vi "MPS_main.vi"() -> ()   [LabVIEW 2021] (continued)
  out "Numeric":i32
  out "Recent File Name":string="MAG_Empty_0,0000010_ug_BatchName"
  in  "name identifier":string="Empty"
  in  "Base path":path=path "D:/HumanImagerData/MPS Data"
  out "Meas Drive IMon Val RMS\nCal BMon":dbl=0.07740384925739274
  in  "Acq Baseline":bool
  in  "CalcConc":bool
  in  "CalcMass":bool
  in  "Sample MetaData Cluster":T1={"Sample Volume (uL)"=10.0, "Sample Mass (ug)"=1e-06, "Sample Conc(mg/mL)"=1e-07, "Sample Temperature (C)"=23.0, "Batch Num"=222.0, "Batch Name"="BatchName", "Solute"="Test", "Solvent"="Water", "Sample Description"="EMPTY"}
  in  "TxRx_Params":T2={"sample rate"=1000000.0, "Tx freq"=23809.52380952381, "Tx amp"=0.05, "Tx cycles\nSpectroscopy"=500.0, "Bias amp"=2.65, "Bias freq"=11.904761904761905, "Receive range"=5.0, "Bias Periods\nMagnetometry"=6.0, "Tx Freq Division Factor"=42.0, "Drive Periods per Bias"=2000.0, "TX harmonics"=[47619.04761904762, 71428.57142857142, 95238.09523809524, 119047.61904761905, 142857.14285714284, 166666.66666666666, 190476.19047619047, 214285.7142857143, 238095.2380952381, 261904.7619047619, 285714.2857142857, 309523.8095238095, 333333.3333333333, 357142.85714285716, 380952.38095238095, 404761.90476190473, 428571.4285714286, 452380.95238095237, 476190.4761904762, 500000.0]} {"TX harmonics" format="%#_6p"}
  in  "Tab Control 2":enum32{"Motor Params", "Motor Move Control"}(tab)=enum."Motor Move Control"
  out "Motor Dir\nT=Fwd":bool=TRUE
  in  "pulse duration (T/2)":dbl=0.0005 format="%#_13p"
  in  "Motor speed":string(combo)="Sixteenth step"
  in  "Sequence to run on start up":string[](array[string])=["Move", "Halt"]
  out "Current Motor State":string="MoveToMax"
  in  "Unsigned Pulses to move":dbl=5.0
  in  "Move-Bed-Back":bool
  in  "Move-Bed-Fwd":bool
  in  "Home then insert sample":bool
  in  "Pulses From Home to Max Sig":dbl=128.0
  in  "Motor Go Home":bool
  out "Empty Bore-BMon-Spec":dbl[](array[numeric])
  out "EmptyBoreBaseline_Mag_BMon":dbl[](array[numeric])
  in  "Toggle fan":bool
  out "Amps Drive Peak":dbl=13.682895644634083
  out "EmptyBoreBaseline_Mag":dbl[](array[numeric])
  out "Samples Per Acquisition":dbl=504000.0
  in  "Run Cal BMon":bool
  out "mT/BMon Volt":dbl=19.366390338753
  out "Meas BMon Val RMS":dbl=0.4592431533931806
  out "Expected mT peak":dbl=8.893882169012155
  in  "Update global variables Button":bool
  in  "stop":bool
  out "current system state":string="Idle"
  out "Main loop has stopped":bool
  in  "Tab Control":T3(tab)=enum."Magnetometry"
  in  "Run Sys Ref Meas":bool
  in  "Use Bias?":bool
  in  "Scanner Description":T4={"Scanner Name"="Test", "Hardware description"="Test", "Preamplifier Used"="INA", "Preamp Gain"=9999.0, "Drive Amplifier"="TDA3255", "Bias Amplifier"="RCF IPS700", "Drive Current Monitor"="Rogowski", "Bias Current Monitor"="ACS-770"}
  in  "Study and Experiment Description":T5={"Study Number"=9999, "Study Name"="Test", "UUID"="93C38C5B-0D33-4591-A951-706E1E8CC347", "GUI Open Time"="2022-04-10_16-04-30", "Notes"="Example"}
  out "3f0 over time":dbl(graph)=3.5778765993993083e-09
  out "Rx FFT":cluster{"f0":dbl, "df":dbl, "magnitude":dbl[]}(graph)={"f0"=0.0, "df"=49.55401387512537, "magnitude"=array[10090 elements]}
  in  "Run Spectroscopy":bool
  in  "Stop Spec":bool
  out "Loop Num":i32=5 format="%.4p"
  in  "Save Spectroscopy":bool=TRUE
  in  "Max Spec Runs":i32=10000
  in  "ms delay":u32=25 format="%#.4p"
  in  "Spec samples\nto crop":dbl=820.0 format="%#_4p"
  out "Spec Time Domain":dbl[][](graph)
  out "f0 over time":dbl(graph)=4.148276400287791e-05
  out "THD":dbl=-79.42517157036677 format="%#_6p"
  out "Expected mT Spec Drive":dbl=9.011999624680417 format="%#_4p"
  out "mean3f0":dbl=3.083839308845972e-09 format="%#_3p"
  out "standard deviation 3f0":dbl=4.1440630531044285e-10 format="%#_4p"
  out "meanf0":dbl=4.1403379240994345e-05 format="%#_3p"
  out "standard deviation f0":dbl=8.05138622723974e-08 format="%#_4p"
  out "Bed moving":bool=TRUE
  in  "ms delay\nevery Spec":u32=50 format="%#.4p"
  in  "Run in-out spec":bool
  out "Expected mT Spec Drive 2":dbl=9.006191537419065 format="%#_4p"
  out "Drive Imon THD 2":dbl=-79.0246761592133 format="%#_6p"
  in  "Spec samples\nto crop_InOut":dbl=820.0 format="%#_4p"
  out "3f0 over time 2":dbl(graph)=9.016336929462854e-10
  out "f0 over time 2":dbl(graph)=6.340842124732096e-07
  out "Loop Num 2":i32=6 format="%.4p"
  out "Spec Time Domain 2":dbl[][](graph)
  out "Rx FFT 2":cluster{"f0":dbl, "df":dbl, "magnitude":dbl[]}(graph)={"f0"=0.0, "df"=49.55401387512537, "magnitude"=array[10090 elements]}
  in  "Num acq per\ncycle":i32=6
  in  "Save Spectroscopy 2":bool=TRUE
  in  "Number of cycles":i32=5
  in  "Pulses in/out":dbl=50.0
  out "Run number":i32=70
  in  "Run Mag":bool
  out "Susceptibility Curves":cluster{"Y":dbl[], "Y":dbl[]}[](graph)
  in  "Save Mag data":bool
  out "Rx Smooth":dbl[](graph)
  out "Sensitivity profile":dbl[][](graph)
  in  "Num Mag Avgs":i32=1 min=1
  out "RunNum":i32
  in  "Pulses in/out 2":dbl=50.0
  in  "ms delay each run":u32
  out "Sample Out":bool
  out "RxEmptyBore-Mag":waveform(dbl)(graph)={"t0"=timestamp(3732466214.765835 s since 1904-01-01), "dt"=9.9999999999997e-07, "Y"=array[504000 elements], "attributes"=variant("NI_ChannelName"=variant(string "H1/ai7"), "NI_UnitDescription"=variant(string "Volts"))}
  out "EmptyBoreBaseline_Spec":dbl[](array[numeric])
  out "RxEmptyBore-Spec":dbl[](graph)
  out "3f0 vs Mass":T6(graph)
  in  "Run DilutionAdd":bool
  in  "ms delay 2":u32=25 format="%#.4p"
  in  "File Name Dilution":string="450ng_Syno"
  in  "Base path 4":path=path "D:/HumanImagerData/MPS Data"
  out "Expected mT Spec Drive 3":dbl=7.493132421986184 format="%#_4p"
  out "THD 2":dbl=-78.20284195000295 format="%#_6p"
  in  "Spec samples\nto crop 3":dbl=820.0 format="%#_4p"
  in  "Num Dil Series Runs":i32=7
  in  "Clear Dilution Array":bool
  out "r^2":dbl format="%.4f"
  in  "Delete Last Meas":bool
  out "Dilution Array\nConc,f0,f3":dbl[][](array[numeric])
  in  "Save Dilution Array":bool
  # "MPS"
  # "FILE SAVING"
  # "NOT WORKING YET"
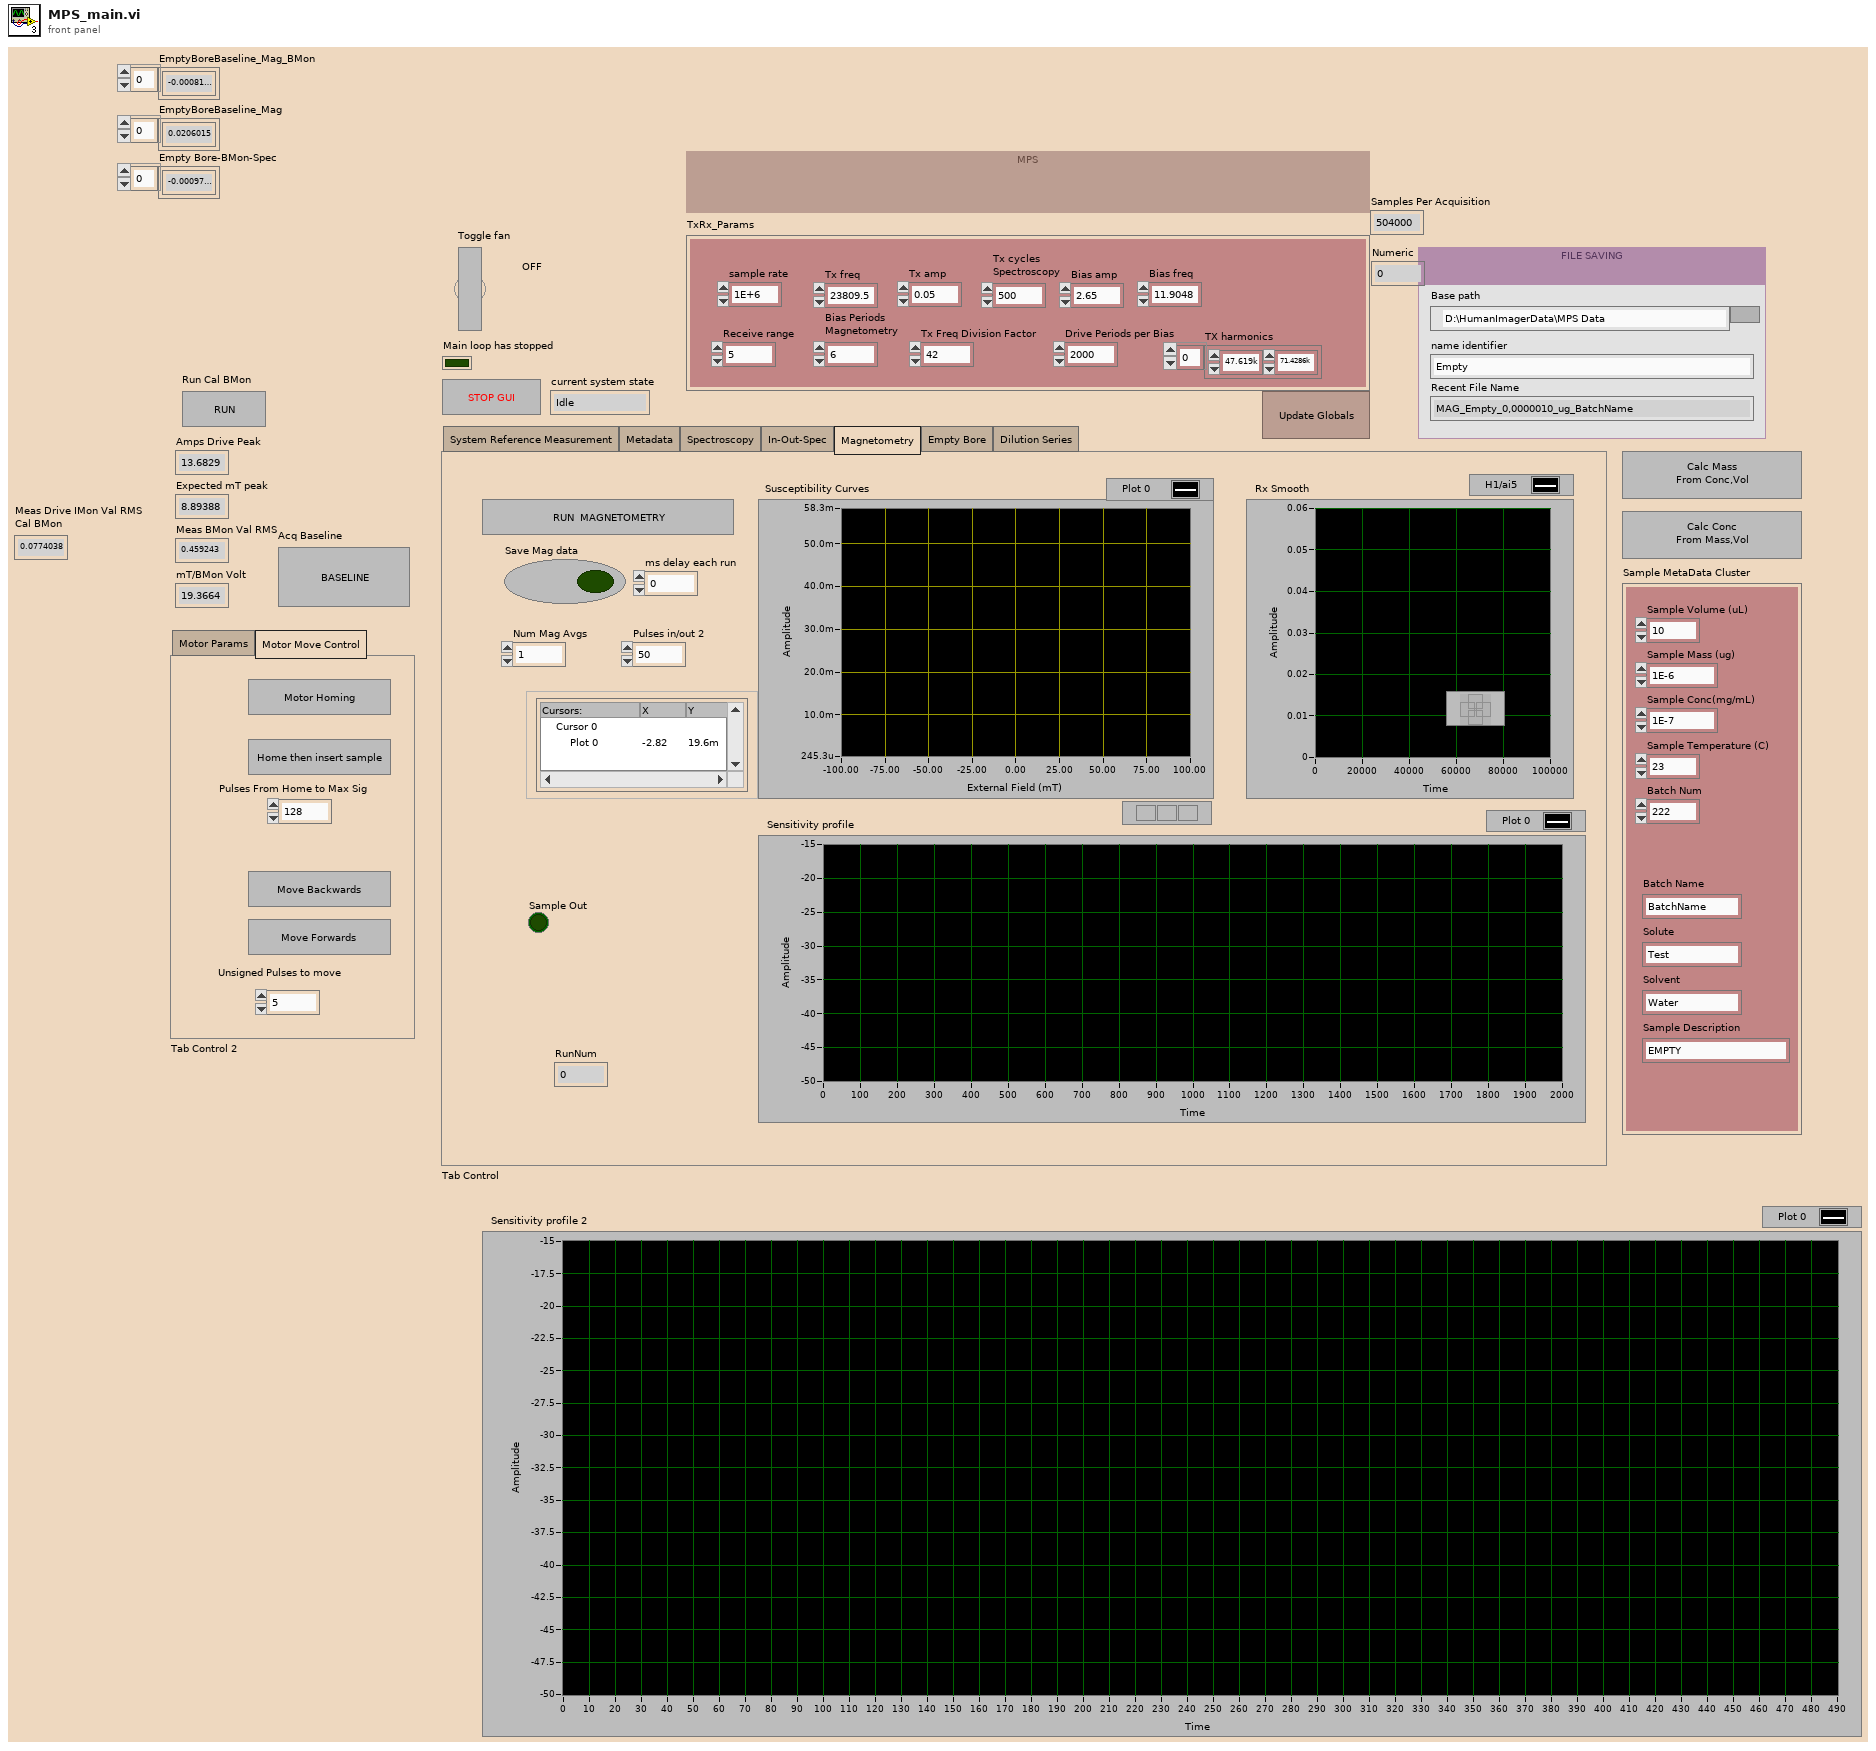
[diagram p1: front panel]
types:
  T1 = cluster{"Sample Volume (uL)":dbl, "Sample Mass (ug)":dbl, "Sample Conc(mg/mL)":dbl, "Sample Temperature (C)":dbl, "Batch Num":dbl, "Batch Name":string, "Solute":string, "Solvent":string, "Sample Description":string}
  T2 = cluster{"sample rate":dbl, "Tx freq":dbl, "Tx amp":dbl, "Tx cycles\nSpectroscopy":dbl, "Bias amp":dbl, "Bias freq":dbl, "Receive range":dbl, "Bias Periods\nMagnetometry":dbl, "Tx Freq Division Factor":dbl, "Drive Periods per Bias":dbl, "TX harmonics":dbl[]}
  T3 = enum32{"System Reference Measurement", "Metadata", "Spectroscopy", "In-Out-Spec", "Magnetometry", "Empty Bore", "Dilution Series"}
  T4 = cluster{"Scanner Name":string, "Hardware description":string, "Preamplifier Used":string, "Preamp Gain":dbl, "Drive Amplifier":string, "Bias Amplifier":string, "Drive Current Monitor":string, "Bias Current Monitor":string}
  T5 = cluster{"Study Number":i64, "Study Name":string, "UUID":string, "GUI Open Time":string, "Notes":string}
  T6 = cluster{"Dilution Array\nConc,f0,f3":dbl[], "Dilution Array\nConc,f0,f3":dbl[]}[]
  T7 = cluster{"sample rate":dbl, "Transmit frequency":dbl, "Transmit amplitude":dbl, "sample rate digital out":dbl, "TX cycles":i32, "sample rate DAQ1":dbl, "Receive frequency":dbl, "Receive range":dbl, "TX harmonics":dbl[]}
  T8 = cluster{"Drive IMon":dbl[], "Rx Time Domain":dbl[], "Rx Empty Bore":dbl[], "BMon":dbl[], "Bias IMon":dbl[], "TF-Corr-MagOverTime":dbl[], "Interpolated Rx TF-Mag":dbl[], "Interpolated Rx TF-Phase":dbl[]}
  T9 = cluster{"slope min":dbl, "slope max":dbl, "intercept min":dbl, "intercept max":dbl}
  T10 = enum32{"none", "input signal", "detected signal", "residual signal"}
  T11 = typedef "NI_AALPro.lvlib/windowTd.ctl" = u32
  T12 = typedef "Tag-dbl.lvlib/))Channel.ctl" = refnum<queue>
  T13 = cluster{"Dilution Array\nConc,f0,f3":dbl[], "Dilution Array\nConc,f0,f3":dbl[]}
  T14 = cluster{"Dilution Array\nConc,f0,f3":dbl[], "Best Linear Fit":dbl[]}
  T15 = cluster{"exported time signal":waveform(dbl), "exported spectrum (dB)":cluster{"f0":dbl, "df":dbl, "dB Spectrum (Hann)":dbl[]}}
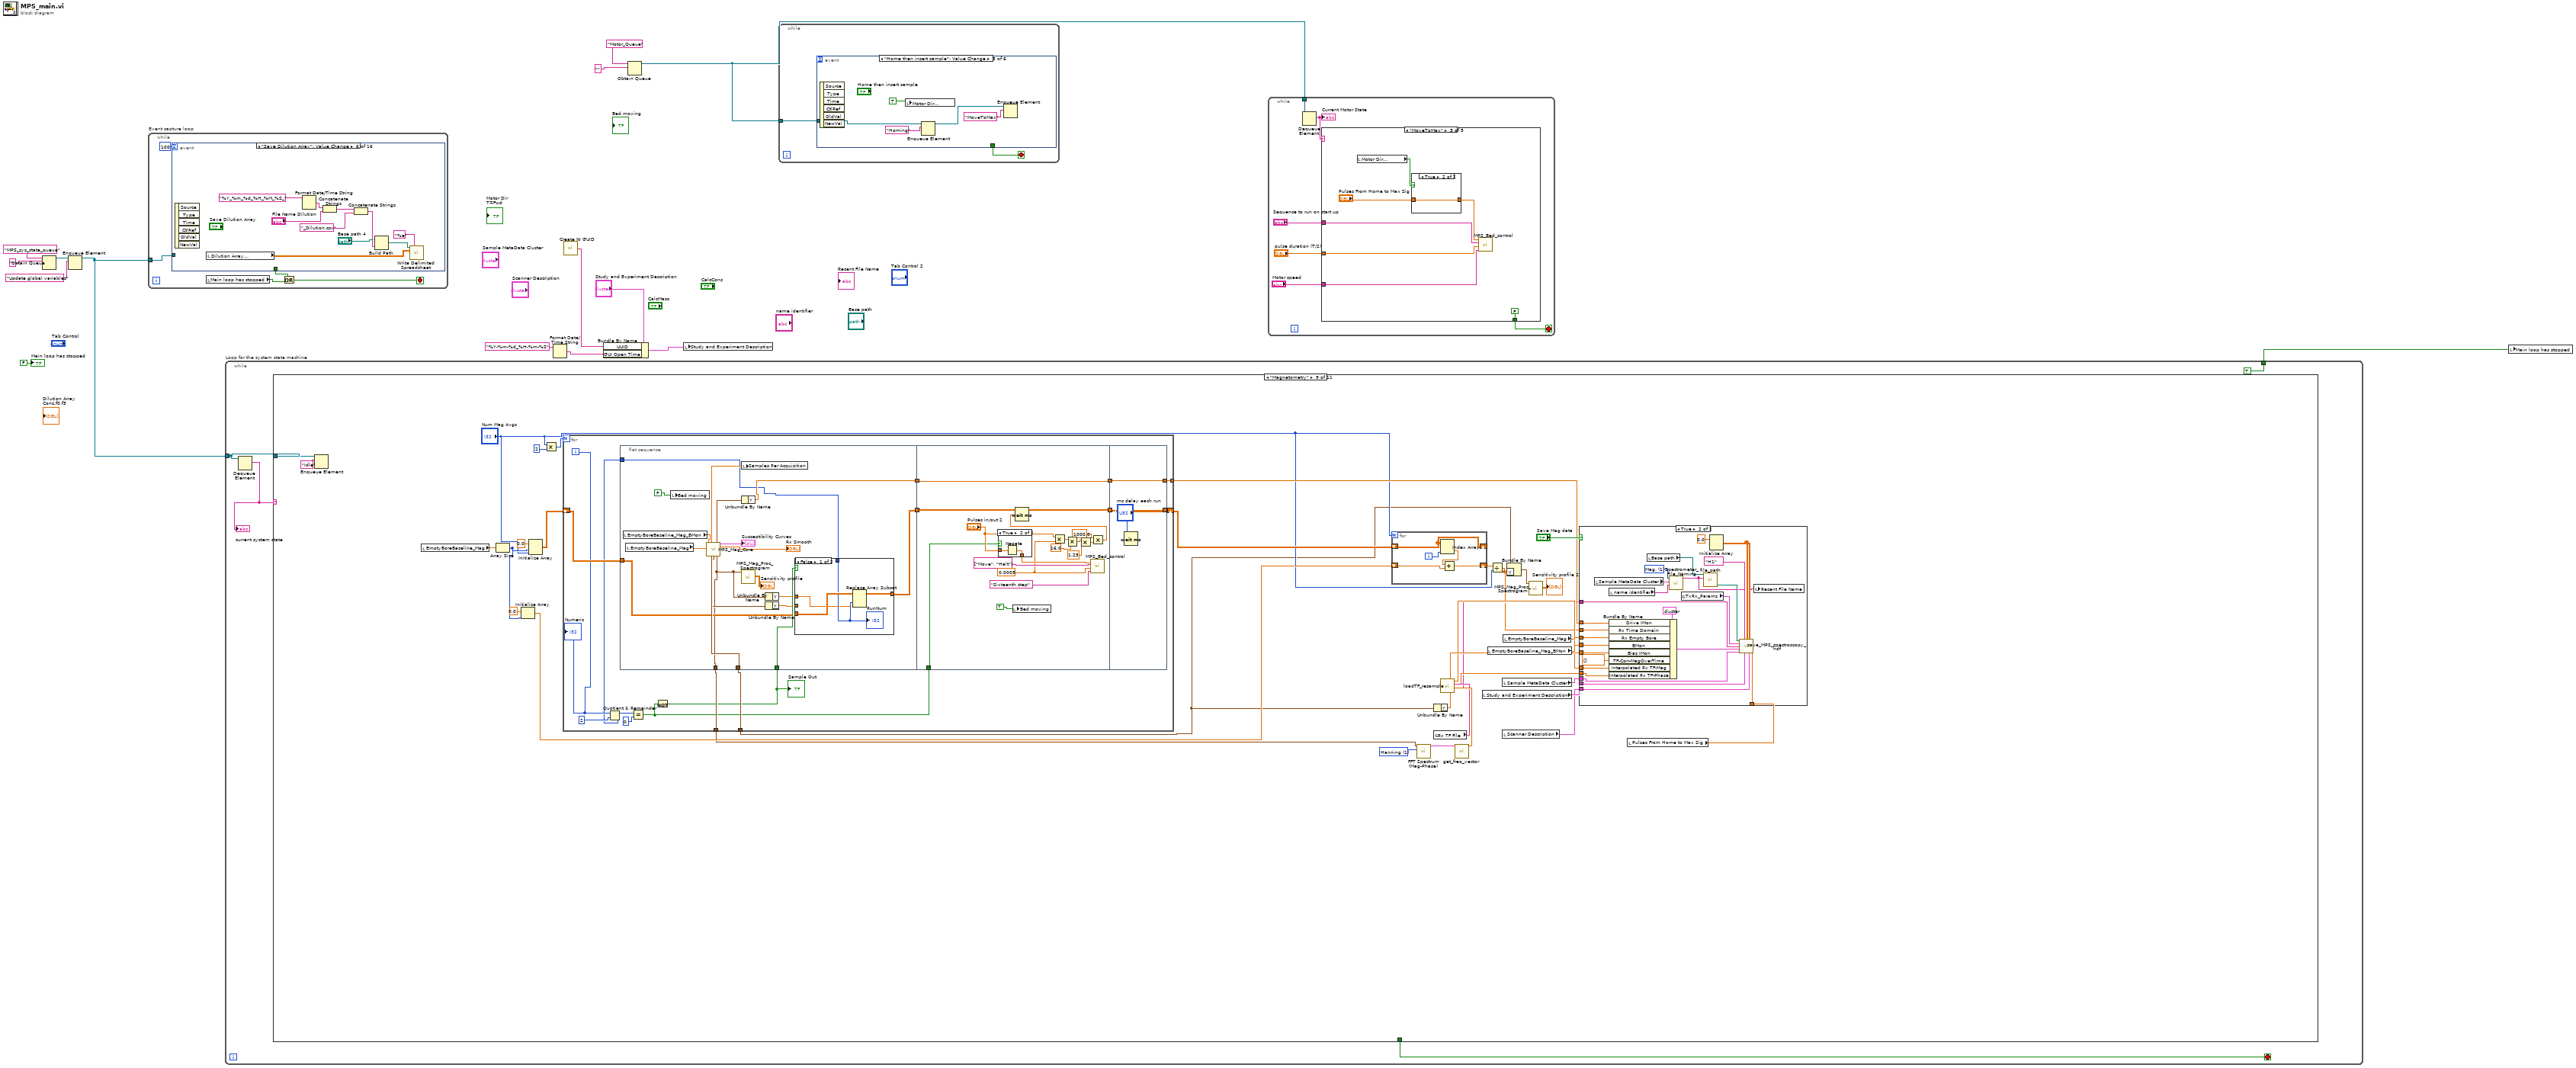
[diagram p0: block diagram]
diagram:
  n1 = Obtain Queue(name (unnamed)="MPS_sys_state_queue", element data type="") -> (queue out=w11:refnum<queue>)  [unwired: 3 in, 2 out]
  n2 = Enqueue Element(queue=w11, element="Update global variables") -> (queue out=w9:refnum<queue>)  [unwired: 2 in, 2 out]
  n3 = while "Event capture loop" {
    tunnel: w9 -> [w19]
    stop <- w16 stop-if-true
    n4 = event shown="[5] \"Save Dilution Array\": Value Change" {
      selector: _ -> [_ _ _ _ _ _ _ _ _ _ _ _ _ _ _ _]
      dyn-events: _ -> [_ _ _ _ _ _ _ _ _ _ _ _ _ _ _ _]
      timeout: 100 -> [_ _ _ _ _ _ _ _ _ _ _ _ _ _ _ _]
      tunnel: w19 -> [_ w22 w24 w26 _ _ _ w66 w68 w70 w72 _ _ _ w93 w96]
      tunnel: [FALSE ("x") _ _ _ _ _ _ _ _ _ _ _ _ _ _ TRUE ("x")] -> w17
      event Timeout {
        n5 = event-data() -> ()  [unwired: 1 in, 3 out]
      }
      event "Run Sys Ref Meas": Value Change {
        n6 = event-data() -> ()  [unwired: 1 in, 6 out]
        n7 = Enqueue Element(queue=w22, element="System Reference Measurement") -> ()  [unwired: 2 in, 3 out]
      }
      event "Run Spectroscopy": Value Change {
        n8 = event-data() -> ()  [unwired: 1 in, 6 out]
        n9 = Enqueue Element(queue=w24, element="Spectroscopy") -> ()  [unwired: 2 in, 3 out]
      }
      event "Run DilutionAdd": Value Change {
        n10 = event-data() -> ()  [unwired: 1 in, 6 out]
        n11 = Enqueue Element(queue=w26, element="Acquire Dilution Data") -> ()  [unwired: 2 in, 3 out]
      }
      event "Clear Dilution Array": Value Change {
        n12 = event-data() -> ()  [unwired: 1 in, 6 out]
        n13 = Initialize Array(0.0 ("element"), 0 ("dimension size"), 3 ("dimension size")) -> (w28:dbl[][])
        n14 = local write "Dilution Array\nConc,f0,f3"(w28) -> ()
        n15 = Index Array(array=w28, index (col)=0 ("disabled index (col)")) -> (element=w35:dbl[])  [unwired: 1 in]
        n16 = Index Array(array=w28, index (col)=2 ("disabled index (col)")) -> (element=w36:dbl[])  [unwired: 1 in]
        n17 = call <vilib>:"Linear Fit.vi"("Y"=w36, "X"=w35) -> ("Best Linear Fit"=w34:dbl[])  [unwired: 9 in, 4 out]
        n18 = Bundle(w35, w36) -> (w32:cluster{dbl[], dbl[]})  [unwired: 1 in]
        n19 = call <vilib>:"Correlation Coefficient (Spearman).vi"("Y"=w36, "X"=w35) -> ()  [unwired: 8 in, 2 out]
        n20 = Bundle(w35, "Best Linear Fit"=w34) -> (w33:cluster{dbl[], "Best Linear Fit":dbl[]})  [unwired: 1 in]
        n21 = Build Array(w33, w32) -> (w31:cluster{dbl[], "Best Linear Fit":dbl[]}[])
        n22 = local write "3f0 vs Mass"(w31) -> ()
      }
      event "Save Dilution Array": Value Change {
        n23 = event-data() -> ()  [unwired: 1 in, 6 out]
        n24 = local read "Dilution Array\nConc,f0,f3"() -> (w41:dbl[][])
        n25 = Format Date/Time String(time format string (%c)="%Y_%m_%d_%H_%M_%S_") -> (date/time string=w47:string)  [unwired: 2 in]
        n26 = Concatenate Strings(w47, "File Name Dilution") -> (w49:string)
        n27 = Concatenate Strings(w49, "_Dilution.csv" ("string")) -> (w48:string)
        n28 = Build Path(base path="Base path 4", name or relative path=w48) -> (appended path=w42:path)
        n29 = call-poly <vilib>:"Write Delimited Spreadsheet.vi"("file path (dialog if empty)"=w42, "format (%.3f)"="%e", "2D data"=w41) -> ()  [unwired: 11 in, 2 out]
      }
      event "Delete Last Meas": Value Change {
        n30 = event-data() -> ()  [unwired: 1 in, 6 out]
        n31 = local read "Dilution Array\nConc,f0,f3"() -> (w65:dbl[][])
        n32 = Array Size(array=w65) -> (size(s)=w64:i32[])
        n33 = Index Array(array=w64, index=0) -> (element=w62:i32)
        n34 = Decrement(x=w62) -> (x-1=w61:i32)
        n35 = Array Subset(array=w65, index (row)=0 ("index"), length (row)=w61, index (col)=0 ("index")) -> (w51:dbl[][])  [unwired: 1 in]
        n36 = local write "Dilution Array\nConc,f0,f3"(w51) -> ()
        n37 = Index Array(array=w51, index (col)=0 ("disabled index (col)")) -> (element=w57:dbl[])  [unwired: 1 in]
        n38 = Index Array(array=w51, index (col)=2 ("disabled index (col)")) -> (element=w58:dbl[])  [unwired: 1 in]
        n39 = call <vilib>:"Linear Fit.vi"("Y"=w58, "X"=w57) -> ("Best Linear Fit"=w56:dbl[])  [unwired: 9 in, 4 out]
        n40 = Bundle(w57, w58) -> (w54:cluster{dbl[], dbl[]})  [unwired: 1 in]
        n41 = call <vilib>:"Correlation Coefficient (Spearman).vi"("Y"=w58, "X"=w57) -> ()  [unwired: 8 in, 2 out]
        n42 = Bundle(w57, "Best Linear Fit"=w56) -> (w55:cluster{dbl[], "Best Linear Fit":dbl[]})  [unwired: 1 in]
        n43 = Build Array(w55, w54) -> (w50:cluster{dbl[], "Best Linear Fit":dbl[]}[])
        n44 = local write "3f0 vs Mass"(w50) -> ()
      }
      event "Run in-out spec": Value Change {
        n45 = event-data() -> ()  [unwired: 1 in, 6 out]
        n46 = Enqueue Element(queue=w66, element="In-Out-Spec") -> ()  [unwired: 2 in, 3 out]
      }
      event "Run Mag": Value Change {
        n47 = event-data() -> ()  [unwired: 1 in, 6 out]
        n48 = Enqueue Element(queue=w68, element="Magnetometry") -> ()  [unwired: 2 in, 3 out]
      }
      event "Acq Baseline": Value Change {
        n49 = event-data() -> ()  [unwired: 1 in, 6 out]
        n50 = Enqueue Element(queue=w70, element="Acquire Empty Bore") -> ()  [unwired: 2 in, 3 out]
      }
      event "Run Cal BMon": Value Change {
        n51 = event-data() -> ()  [unwired: 1 in, 6 out]
        n52 = Enqueue Element(queue=w72, element="Cal_BMon") -> ()  [unwired: 2 in, 3 out]
      }
      event "CalcMass": Value Change {
        n53 = event-data() -> ()  [unwired: 1 in, 6 out]
        n54 = local read "Sample MetaData Cluster"() -> (w78:T1)
        n55 = Unbundle By Name(w78) -> ("Sample Volume (uL)"=w77:dbl, "Sample Conc(mg/mL)"=w76:dbl)
        n56 = Multiply(x=w77, y=w76) -> (x*y=w74:dbl)
        n57 = Bundle By Name(cluster=w78, "Sample Mass (ug)"=w74) -> (w75:T1)
        n58 = local write "Sample MetaData Cluster"(w75) -> ()
      }
      event "CalcConc": Value Change {
        n59 = event-data() -> ()  [unwired: 1 in, 6 out]
        n60 = local read "Sample MetaData Cluster"() -> (w83:T1)
        n61 = Unbundle By Name(w83) -> ("Sample Mass (ug)"=w82:dbl, "Sample Volume (uL)"=w81:dbl)
        n62 = Divide(x=w82, y=w81) -> (x/y=w79:dbl)
        n63 = Bundle By Name(cluster=w83, "Sample Conc(mg/mL)"=w79) -> (w80:T1)
        n64 = local write "Sample MetaData Cluster"(w80) -> ()
      }
      event "Toggle fan": Value Change {
        n65 = event-data() -> ()  [unwired: 1 in, 6 out]
        n66 = global read "MPS_global_variables.vi" "Fan Control Line"() -> (w88:tag)
        n67 = call-poly <vilib>:"DAQmx Create Virtual Channel.vi"("lines"=w88) -> ("task out"=w90:refnum<k21>, "error out"=w91:errorcluster)  [unwired: 13 in]
        n68 = call-poly <vilib>:"DAQmx Write.vi"("task/channels in"=w90, "data"="Toggle fan", "error in"=w91) -> ("task out"=w87:refnum<k21>, "error out"=w86:errorcluster)  [unwired: 10 in, 1 out]
        n69 = call <vilib>:"DAQmx Stop Task.vi"("task/channels in"=w87, "error in"=w86) -> ("task out"=w85:refnum<k21>, "error out"=w84:errorcluster)  [unwired: 12 in]
        n70 = call <vilib>:"DAQmx Clear Task.vi"("task in"=w85, "error in"=w84) -> ()  [unwired: 13 in, 1 out]
      }
      event "Update global variables Button": Value Change {
        n71 = event-data() -> ()  [unwired: 1 in, 6 out]
        n72 = Enqueue Element(queue=w93, element="Update global variables") -> ()  [unwired: 2 in, 3 out]
      }
      event "stop": Value Change {
        n73 = event-data() -> ()  [unwired: 1 in, 6 out]
        n74 = Enqueue Element(queue=w96, element="Halt") -> ()  [unwired: 2 in, 3 out]
      }
    }
    n75 = local read "Main loop has stopped"() -> (w18:bool)
    n76 = Or(x=w17, y=w18) -> (x .or. y?=w16:bool)
  }
  n77 = while "Loop for the system state machine" {
    tunnel: w9 -> [w98]
    tunnel: [TRUE ("Main loop has stopped")] -> w12
    stop <- w100 stop-if-true
    n78 = Dequeue Element(queue=w98) -> (element=w97:string)  [unwired: 2 in, 3 out]
    "current system state" <- w97
    n79 = case shown="\"Magnetometry\"" w97 {
      tunnel: [_ _ _ _ _ _ _ _ _ _ TRUE] -> w100
      tunnel: w98 -> [_ w103 w132 w178 w226 w325 w393 _ w560 w654 _]
      frame "Idle", Default {
      }
      frame "Update global variables" {
        n80 = Enqueue Element(queue=w103, element="Idle") -> ()  [unwired: 2 in, 3 out]
        n81 = flat-sequence {
          tunnel: [w108] -> w101
          tunnel: w101 -> [w113]
          frame #0 {
            n82 = Unbundle By Name("TxRx_Params") -> ("sample rate"=w112:dbl, "Tx Freq Division Factor"=w110:dbl, "Drive Periods per Bias"=w109:dbl)
            n83 = Divide(x=w112, y=w110) -> (x/y=w106:dbl)
            n84 = Divide(x=w106, y=w109) -> (x/y=w111:dbl)
            n85 = Multiply(x=w106, y=dbl[] [2.0, 3.0, 4.0, 5.0, 6.0, 7.0, 8.0, 9.0, 10.0, 11.0, 12.0, 13.0, 14.0, 15.0, 16.0, 17.0, 18.0, 19.0, 20.0, 21.0]) -> (x*y=w104:dbl[])
            n86 = Bundle By Name(cluster="TxRx_Params", "Tx freq"=w106, "Bias freq"=w111, "TX harmonics"=w104) -> (w108:T2)
            n87 = global write "MPS_global_variables.vi" "TxRx_Params"(w108) -> ()
          }
          frame #1 {
            n88 = local write "TxRx_Params"(w113) -> ()
          }
        }
      }
      frame "System Reference Measurement" {
        w124 = T11 1 items=["Rectangle"=0, "Hanning"=1, "Hamming"=2, "Blackman-Harris"=3, "Exact Blackman"=4, "Blackman"=5, "Flat Top"=6, "4 Term B-Harris "=7, "7 Term B-Harris"=8, "Low Sidelobe"=9, "Blackman Nuttall"=11, "Triangle"=30, "Bartlett-Hanning"=31, "Bohman"=32, "Parzen"=33, "Welch"=34, "Kaiser"=60, "Dolph-Chebyshev"=61, "Gaussian"=62] ("window")
        # "Data queue"
        n89 = global read "MPS_global_variables.vi" "TxRx_Params"() -> (w121:T2)
        n90 = Enqueue Element(queue=w132, element="Idle") -> ()  [unwired: 2 in, 3 out]
        n91 = Unbundle By Name(w121) -> ("Bias Periods\nMagnetometry"=w117:dbl, "sample rate"=w120:dbl, "Bias freq"=w119:dbl)
        n92 = Divide(x=w120, y=w119) -> (x/y=w118:dbl)
        n93 = Multiply(x=w117, y=w118) -> (x*y=w116:dbl)
        n94 = Round To Nearest(number=w116) -> (nearest integer value=w115:dbl)
        n95 = local write "Samples Per Acquisition"(w115) -> ()
        n96 = Initialize Array(waveform(dbl) {"t0"=timestamp(0 s since 1904-01-01), "dt"=1.0, "Y"=[]} ("Waveform")) -> (w126:waveform(dbl)[])  [unwired: 1 in]
        n97 = Obtain Queue(element data type=w126) -> (queue out=w125:refnum<queue>)  [unwired: 4 in, 2 out]
        n98 = Obtain Queue(element data type=w126) -> (queue out=w127:refnum<queue>)  [unwired: 4 in, 2 out]
        n99 = call <extravilib>:"Write.vi"("element"=1 ("number of readouts")) -> ("channel"=w128:T12)  [unwired: 1 out]
        n100 = flat-sequence {
          tunnel: w127 -> [w138]
          tunnel: [w137] -> w129
          tunnel: w128 -> [w141]
          tunnel: w125 -> [w137]
          tunnel: [w136] -> w122
          tunnel: w115 -> [w135]
          tunnel: ["Use Bias?"] -> w114
          tunnel: w129 -> [w151]
          tunnel: w128 -> [w150]
          tunnel: [w142] -> _
          tunnel: w115 -> [w146]
          tunnel: w114 -> [w145]
          frame #0 {
            (unwired) TRUE
            n101 = Dequeue Element(queue=w138) -> (element=w139:waveform(dbl)[])  [unwired: 2 in, 3 out]
            n102 = Index Array(array=w139, index=0) -> (element=w136:waveform(dbl))
            n103 = call "MPS_transmit_receive.vi"("samples per readout"=w135, "Use Bias?"="Use Bias?", "channel input for max readouts"=w141) -> ()  [unwired: 9 in]
          }
          frame #1 {
            (unwired) FALSE
            n104 = Dequeue Element(queue=w151) -> (element=w147:waveform(dbl)[])  [unwired: 2 in, 3 out]
            n105 = global read "MPS_global_variables.vi" "Volts Per Amp\nBias"() -> (w144:dbl)
            n106 = call "MPS_transmit_receive.vi"("samples per readout"=w146, "Use Bias?"=w145, "channel input for max readouts"=w150) -> ()  [unwired: 9 in]
            n107 = Index Array(array=w147, index=1) -> ()  [unwired: 1 out]
            n108 = Index Array(array=w147, index=0) -> (element=w143:waveform(dbl))
            n109 = Divide(x=w143, y=w144) -> (x/y=w142:waveform(dbl))
          }
        }
        n110 = call-poly <vilib>:"Get Waveform Time Array.vi"("waveform in"=w122) -> ()  [unwired: 9 in, 2 out]
        n111 = call-poly <vilib>:"FFT Spectrum (Mag-Phase).vi"("window"=w124, "time signal"=w122) -> ("magnitude"=w123:cluster{"f0":dbl, "df":dbl, "magnitude":dbl[]})  [unwired: 5 in, 4 out]
        n112 = Complex To Polar(r * e^(i*theta)=w123) -> ()  [unwired: 2 out]
      }
      frame "Cal_BMon" {
        w160 = waveform(dbl) {"t0"=timestamp(0 s since 1904-01-01), "dt"=1.0, "Y"=[]} ("Waveform")
        # "Acquire Drive IMon"
        # "Acquire BMon"
        # "Data queue"
        n113 = Enqueue Element(queue=w178, element="Idle") -> ()  [unwired: 2 in, 3 out]
        n114 = global read "MPS_global_variables.vi" "TxRx_Params"() -> (w168:T2)
        n115 = Obtain Queue(element data type=w160) -> (queue out=w179:refnum<queue>)  [unwired: 4 in, 2 out]
        n116 = Obtain Queue(element data type=w160) -> (queue out=w180:refnum<queue>)  [unwired: 4 in, 2 out]
        n117 = call <extravilib>:"Write.vi"("element"=1 ("number of readouts")) -> ("channel"=w181:T12)  [unwired: 1 out]
        n118 = Unbundle By Name(w168) -> ("Tx cycles\nSpectroscopy"=w164:dbl, "sample rate"=w167:dbl, "Tx freq"=w166:dbl)
        n119 = flat-sequence {
          tunnel: w180 -> [w187]
          tunnel: [w190] -> w184
          tunnel: w181 -> [w191]
          tunnel: w179 -> [w190]
          tunnel: w162 -> [w188]
          tunnel: [w185] -> w159
          tunnel: w184 -> [w194]
          tunnel: w181 -> [w197]
          tunnel: w162 -> [w195]
          tunnel: [w192] -> w158
          frame #0 {
            n120 = Dequeue Element(queue=w187) -> (element=w185:waveform(dbl))  [unwired: 2 in, 3 out]
            n121 = call "MPS_transmit_receive.vi"("samples per readout"=w188, "Use Bias?"=FALSE, "InputChans"=enum16{"Rx", "BiasIMon", "TxIMon", "BMon"}."TxIMon", "channel input for max readouts"=w191, "Measurement Queue"=w187) -> ()  [unwired: 7 in]
          }
          frame #1 {
            n122 = Dequeue Element(queue=w194) -> (element=w192:waveform(dbl))  [unwired: 2 in, 3 out]
            n123 = call "MPS_transmit_receive.vi"("samples per readout"=w195, "Use Bias?"=FALSE, "InputChans"=enum16{"Rx", "BiasIMon", "TxIMon", "BMon"}."BMon", "channel input for max readouts"=w197, "Measurement Queue"=w194) -> ()  [unwired: 7 in]
          }
        }
        n124 = Divide(x=w167, y=w166) -> (x/y=w165:dbl)
        n125 = Multiply(x=w164, y=w165) -> (x*y=w163:dbl)
        n126 = Round To Nearest(number=w163) -> (nearest integer value=w162:dbl)
        "Samples Per Acquisition" <- w162
        n127 = global read "MPS_global_variables.vi" "TxRx_Params"() -> (w172:T2)
        n128 = Unbundle By Name(w172) -> ("Tx freq"=w171:dbl)
        n129 = call-poly <vilib>:"FFT Spectrum (Mag-Phase).vi"("time signal"=w159) -> ("phase"=w175:cluster{"f0":dbl, "df":dbl, "phase":dbl[]}, "magnitude"=w174:cluster{"f0":dbl, "df":dbl, "magnitude":dbl[]})  [unwired: 6 in, 3 out]
        n130 = call-poly <vilib>:"FFT Spectrum (Mag-Phase).vi"("time signal"=w158) -> ("phase"=w176:cluster{"f0":dbl, "df":dbl, "phase":dbl[]}, "magnitude"=w177:cluster{"f0":dbl, "df":dbl, "magnitude":dbl[]})  [unwired: 6 in, 3 out]
        n131 = Bundle By Name(cluster=T7 {"sample rate"=1000000.0, "Transmit frequency"=25000.0, "Transmit amplitude"=1.577, "sample rate digital out"=40000.0, "TX cycles"=600, "sample rate DAQ1"=1000000.0, "Receive frequency"=75000.0, "Receive range"=1.0, "TX harmonics"=[50000.0, 75000.0, 100000.0, 125000.0, 150000.0, 175000.0, 200000.0, 225000.0]} ("TxRxParams"), "Transmit frequency"=w171, "Receive frequency"=w171) -> (w170:T7)
        n132 = call "determine_harmonics.vi"("FFT magnitude"=w174, "FFT phase"=w175, "TxRxParams"=w170) -> ("RX magnitude"=w161:dbl)  [unwired: 11 in, 5 out]
        "Meas Drive IMon Val RMS\nCal BMon" <- w161
        n133 = call "determine_harmonics.vi"("FFT magnitude"=w177, "FFT phase"=w176, "TxRxParams"=w170) -> ("RX magnitude"=w153:dbl)  [unwired: 11 in, 5 out]
        "Meas BMon Val RMS" <- w153
        n134 = call "MPS_Drive_ImonScale.vi"("Drive IMon FFT Mag RMS"=w161) -> ("Amps Drive Peak"=→"Amps Drive Peak":dbl, "Expected mT Peak"=w156:dbl)  [unwired: 9 in]
        "Expected mT peak" <- w156
        n135 = Square Root(x=2.0) -> (sqrt(x)=w155:dbl)
        n136 = Multiply(x=w153, y=w155) -> (x*y=w152:dbl)
        n137 = Divide(x=w156, y=w152) -> (x/y=w169:dbl)
        "mT/BMon Volt" <- w169
        n138 = global write "MPS_global_variables.vi" "mT/BMon Volt"(w169) -> ()
      }
      frame "Spectroscopy" {
        n139 = Enqueue Element(queue=w226, element="Idle") -> ()  [unwired: 2 in, 3 out]
        n140 = Initialize Array(0.0 ("element"), 0 ("dimension size"), 9 ("dimension size")) -> (w216:dbl[][])
        n141 = Initialize Array(0.0 ("element"), 0 ("dimension size"), 9 ("dimension size")) -> (w221:dbl[][])
        n142 = while {
          tunnel: [w293] -> w225
          tunnel: [w292] -> w224
          shift-right: [w290] -> w205
          shift-left: w221 -> [w291]
          tunnel: w216 -> [w289]
          tunnel: [w288] -> w215
          tunnel: [w276] -> w214
          tunnel: [w270] -> w213
          tunnel: [w262] -> w203
          tunnel: [w257] -> w202
          tunnel: [w255] -> w201
          tunnel: [w256] -> w200
          i -> [w287]
          stop <- w283 stop-if-true
          w272 = T11 1 items=["Rectangle"=0, "Hanning"=1, "Hamming"=2, "Blackman-Harris"=3, "Exact Blackman"=4, "Blackman"=5, "Flat Top"=6, "4 Term B-Harris "=7, "7 Term B-Harris"=8, "Low Sidelobe"=9, "Blackman Nuttall"=11, "Triangle"=30, "Bartlett-Hanning"=31, "Bohman"=32, "Parzen"=33, "Welch"=34, "Kaiser"=60, "Dolph-Chebyshev"=61, "Gaussian"=62] ("window")
          n143 = local read "RxEmptyBore-Spec"() -> (w282:dbl[])
          n144 = call "MPS_Spectroscopy_Core.vi"("EmptyBoreBaseline_Spec"=w282, "ms delay"="ms delay", "Spec samples\nto crop"="Spec samples\nto crop") -> ("f0 Complex"=w266:cdb, "phase f1-f9"=w278:dbl[], "TF Corr Rx FFT Mag"=→"Rx FFT":cluster{"f0":dbl, "df":dbl, "magnitude":dbl[]}, "Spec Waveform Baseline Sub"=w271:waveform(dbl), "Drive IMon"=w277:waveform(dbl), "3f0 Complex"=w269:cdb, "mag f1-f9"=w279:dbl[], "Expected mT Spec Drive"=→"Expected mT Spec Drive":dbl, "TF Corrected\nMagnetization over time"=w265:waveform(dbl)[], "Spec Time Domain"=→"Spec Time Domain":dbl[][], "THD"=→"THD":dbl)  [unwired: 2 in, 4 out]
          n145 = Complex To Polar(r * e^(i*theta)=w266) -> (r=→"f0 over time":dbl)  [unwired: 1 out]
          n146 = Complex To Polar(r * e^(i*theta)=w269) -> (r=→"3f0 over time":dbl)  [unwired: 1 out]
          n147 = Unbundle By Name(w277) -> ("Y"=w276:dbl[])
          n148 = Unbundle By Name(w271) -> ("Y"=w270:dbl[])
          n149 = Index Array(array=w265, index=1) -> (element=w263:waveform(dbl))
          n150 = Unbundle By Name(w263) -> ("Y"=w262:dbl[])
          n151 = call-poly <vilib>:"FFT Spectrum (Mag-Phase).vi"("window"=w272, "time signal"=w271) -> ("magnitude"=w260:cluster{"f0":dbl, "df":dbl, "magnitude":dbl[]})  [unwired: 5 in, 4 out]
          n152 = global read "MPS_global_variables.vi" "Rx TF File"() -> (w259:string)
          n153 = call "get_freq_vector.vi"("FFT magnitude"=w260) -> ("Freq array"=w261:dbl[])  [unwired: 10 in]
          n154 = call "loadTF_resample.vi"("desired freqs"=w261, "mat file name"=w259) -> ("TF units from loaded file"=w255:string, "output TF phase"=w256:dbl[], "output TF mag"=w257:dbl[])  [unwired: 7 in]
          n155 = Greater Or Equal?(x=w287, y="Max Spec Runs") -> (x >= y?=w284:bool)
          n156 = Or(x="Stop Spec", y=w284) -> (x .or. y?=w283:bool)
          n157 = local read "Empty Bore-BMon-Spec"() -> (w292:dbl[])
          n158 = local read "RxEmptyBore-Spec"() -> (w293:dbl[])
          n159 = Insert Into Array(array=w291, index (row)=w287, new element=w279) -> (w290:dbl[][])  [unwired: 1 in]
          n160 = Insert Into Array(array=w289, index (row)=w287, new element=w278) -> (w288:dbl[][])  [unwired: 1 in]
          "Loop Num" <- w287
        }
        n161 = Index Array(array=w205, index (col)=2 ("index")) -> (element=w212:dbl[])  [unwired: 1 in]